vi "HFRR ADV v041.vi"() -> ()   [LabVIEW 2025] (continued)
          }
        }
        n1338 = local write "CAMERA ROI MAX TEMP"(TRUE ("CAMERA ROI MAX TEMP")) -> ()
      }
      frame "Adv Scar" {
        n1339 = local read "CAMERA ROI MIN TEMP"() -> (w1648:bool)
        n1340 = case shown="True" "LIVE FEED MAX TEMP" {
          selector: "LIVE FEED MAX TEMP" -> [_ w1669]
          frame False {
          }
          frame True {
            n1341 = Not(x=w1669) -> (.not. x?=w1668:bool)
            n1342 = local write "LIVE FEED MAX TEMP"(w1668) -> ()
            n1343 = call "CAMERA LIVE FEED FGV.vi"("Enum - Menu"=CAMERA_LIVE_FEED_ENUM."CAMERA RESTORE") -> ("error out"=w1659:errorcluster)  [unwired: 9 in, 1 out]
            n1344 = Type Cast(type=30, x=0) -> (*(type *) &x=w1663:i32)
            n1345 = Add(x=w1663, y=48) -> (x+y=w1664:i32)
            n1346 = call "CAMERA LIVE FEED FGV.vi"("Enum - Menu"=CAMERA_LIVE_FEED_ENUM."CAMERA MODE SET", "error in (no error)"=w1659, "CAMERA MODE"=w1664) -> ("error out"=w1656:errorcluster)  [unwired: 7 in, 1 out]
            n1347 = call "CAMERA LIVE FEED FGV.vi"("Enum - Menu"=CAMERA_LIVE_FEED_ENUM."CAMERA GRAY", "error in (no error)"=w1656) -> ("error out"=w1655:errorcluster)  [unwired: 8 in, 1 out]
            n1348 = call "LIST FILE NAMES.vi"("error in (no error)"=w1655) -> ("error out"=w1665:errorcluster, "filenames"=w1666:string[])  [unwired: 9 in]
            n1349 = property on="FILE 3" class="CmbBox"(error in=w1665, "Strings[]"=w1666) -> ()  [unwired: 1 in, 2 out]
          }
        }
        n1350 = case shown="True" w1648 {
          selector: w1648 -> [_ w1654]
          frame False {
          }
          frame True {
            n1351 = Not(x=w1654) -> (.not. x?=w1653:bool)
            n1352 = local write "CAMERA ROI MIN TEMP"(w1653) -> ()
            n1353 = call "IMAGE ANALYSIS.vi"("Enum"=POST_ANALYSIS_ENUM."MINIMIZE UI") -> ()  [unwired: 9 in, 2 out]
          }
        }
        n1354 = local write "CAMERA ROI MAX TEMP"(TRUE ("CAMERA ROI MAX TEMP")) -> ()
        "LIVE FEED MIN TEMP" <- TRUE ("LIVE FEED MIN TEMP")
      }
      frame "Adv Scar Report" {
        n1355 = local read "CAMERA ROI MAX TEMP"() -> (w1670:bool)
        n1356 = local read "LIVE FEED MIN TEMP"() -> (w1672:bool)
        n1357 = local write "LIVE FEED MAX TEMP"(TRUE ("LIVE FEED MAX TEMP")) -> ()
        n1358 = case shown="True" w1672 {
          selector: w1672 -> [_ w1681]
          frame False {
          }
          frame True {
            n1359 = Not(x=w1681) -> (.not. x?=w1680:bool)
            n1360 = local write "LIVE FEED MIN TEMP"(w1680) -> ()
            n1361 = call "CAMERA LIVE FEED FGV.vi"("Enum - Menu"=CAMERA_LIVE_FEED_ENUM."CAMERA MINIMIZE") -> ()  [unwired: 9 in, 2 out]
          }
        }
        n1362 = case shown="True" w1670 {
          selector: w1670 -> [_ w1678]
          frame False {
          }
          frame True {
            n1363 = Not(x=w1678) -> (.not. x?=w1676:bool)
            n1364 = local write "CAMERA ROI MAX TEMP"(w1676) -> ()
            n1365 = call "IMAGE ANALYSIS.vi"("Enum"=POST_ANALYSIS_ENUM."SHOW UI") -> ("error out"=w1675:errorcluster)  [unwired: 9 in, 1 out]
            n1366 = call "LIST FILE NAMES.vi"("error in (no error)"=w1675) -> ("filenames"=w1674:string[])  [unwired: 9 in, 1 out]
            n1367 = property on="Test File List :" class="CmbBox"("Strings[]"=w1674) -> ()  [unwired: 2 in, 2 out]
          }
        }
        n1368 = local write "CAMERA ROI MIN TEMP"(TRUE ("CAMERA ROI MIN TEMP")) -> ()
      }
      frame "Compare Files" {
        n1369 = local read "LIVE FEED MIN TEMP"() -> (w1684:bool)
        n1370 = local write "LIVE FEED MAX TEMP"(TRUE ("LIVE FEED MAX TEMP")) -> ()
        n1371 = local read "CAMERA ROI MIN TEMP"() -> (w1682:bool)
        n1372 = case shown="True" w1684 {
          selector: w1684 -> [_ w1691]
          frame False {
          }
          frame True {
            n1373 = Not(x=w1691) -> (.not. x?=w1690:bool)
            n1374 = local write "LIVE FEED MIN TEMP"(w1690) -> ()
            n1375 = call "CAMERA LIVE FEED FGV.vi"("Enum - Menu"=CAMERA_LIVE_FEED_ENUM."CAMERA MINIMIZE") -> ()  [unwired: 9 in, 2 out]
          }
        }
        n1376 = case shown="True" w1682 {
          selector: w1682 -> [_ w1688]
          frame False {
          }
          frame True {
            n1377 = Not(x=w1688) -> (.not. x?=w1687:bool)
            n1378 = local write "CAMERA ROI MIN TEMP"(w1687) -> ()
            n1379 = call "IMAGE ANALYSIS.vi"("Enum"=POST_ANALYSIS_ENUM."MINIMIZE UI") -> ()  [unwired: 9 in, 2 out]
          }
        }
        n1380 = local write "CAMERA ROI MAX TEMP"(TRUE ("CAMERA ROI MAX TEMP")) -> ()
      }
      frame "About" {
        n1381 = local read "LIVE FEED MIN TEMP"() -> (w1694:bool)
        n1382 = local write "LIVE FEED MAX TEMP"(TRUE ("LIVE FEED MAX TEMP")) -> ()
        n1383 = local read "CAMERA ROI MIN TEMP"() -> (w1693:bool)
        n1384 = case shown="True" w1694 {
          selector: w1694 -> [_ w1701]
          frame False {
          }
          frame True {
            n1385 = Not(x=w1701) -> (.not. x?=w1700:bool)
            n1386 = local write "LIVE FEED MIN TEMP"(w1700) -> ()
            n1387 = call "CAMERA LIVE FEED FGV.vi"("Enum - Menu"=CAMERA_LIVE_FEED_ENUM."CAMERA MINIMIZE") -> ()  [unwired: 9 in, 2 out]
          }
        }
        n1388 = case shown="True" w1693 {
          selector: w1693 -> [_ w1698]
          frame False {
          }
          frame True {
            n1389 = Not(x=w1698) -> (.not. x?=w1697:bool)
            n1390 = local write "CAMERA ROI MIN TEMP"(w1697) -> ()
            n1391 = call "IMAGE ANALYSIS.vi"("Enum"=POST_ANALYSIS_ENUM."MINIMIZE UI") -> ()  [unwired: 9 in, 2 out]
          }
        }
        n1392 = local write "CAMERA ROI MAX TEMP"(TRUE ("CAMERA ROI MIN TEMP")) -> ()
      }
      frame "Advance" {
        n1393 = local read "LIVE FEED MIN TEMP"() -> (w1704:bool)
        n1394 = local write "LIVE FEED MAX TEMP"(TRUE ("LIVE FEED MAX TEMP")) -> ()
        n1395 = local read "CAMERA ROI MIN TEMP"() -> (w1702:bool)
        n1396 = case shown="True" w1704 {
          selector: w1704 -> [_ w1711]
          frame False {
          }
          frame True {
            n1397 = Not(x=w1711) -> (.not. x?=w1710:bool)
            n1398 = local write "LIVE FEED MIN TEMP"(w1710) -> ()
            n1399 = call "CAMERA LIVE FEED FGV.vi"("Enum - Menu"=CAMERA_LIVE_FEED_ENUM."CAMERA MINIMIZE") -> ()  [unwired: 9 in, 2 out]
          }
        }
        n1400 = local write "CAMERA ROI MAX TEMP"(TRUE ("CAMERA ROI MAX TEMP")) -> ()
        n1401 = case shown="True" w1702 {
          selector: w1702 -> [_ w1708]
          frame False {
          }
          frame True {
            n1402 = Not(x=w1708) -> (.not. x?=w1707:bool)
            n1403 = local write "CAMERA ROI MIN TEMP"(w1707) -> ()
            n1404 = call "IMAGE ANALYSIS.vi"("Enum"=POST_ANALYSIS_ENUM."MINIMIZE UI") -> ()  [unwired: 9 in, 2 out]
          }
        }
      }
      frame "Mooha" {
        n1405 = local read "LIVE FEED MIN TEMP"() -> (w1714:bool)
        n1406 = local write "LIVE FEED MAX TEMP"(TRUE ("LIVE FEED MAX TEMP")) -> ()
        n1407 = local read "CAMERA ROI MIN TEMP"() -> (w1712:bool)
        n1408 = case shown="True" w1714 {
          selector: w1714 -> [_ w1721]
          frame False {
          }
          frame True {
            n1409 = Not(x=w1721) -> (.not. x?=w1720:bool)
            n1410 = local write "LIVE FEED MIN TEMP"(w1720) -> ()
            n1411 = call "CAMERA LIVE FEED FGV.vi"("Enum - Menu"=CAMERA_LIVE_FEED_ENUM."CAMERA MINIMIZE") -> ()  [unwired: 9 in, 2 out]
          }
        }
        n1412 = local write "CAMERA ROI MAX TEMP"(TRUE ("CAMERA ROI MAX TEMP")) -> ()
        n1413 = case shown="True" w1712 {
          selector: w1712 -> [_ w1718]
          frame False {
          }
          frame True {
            n1414 = Not(x=w1718) -> (.not. x?=w1717:bool)
            n1415 = local write "CAMERA ROI MIN TEMP"(w1717) -> ()
            n1416 = call "IMAGE ANALYSIS.vi"("Enum"=POST_ANALYSIS_ENUM."MINIMIZE UI") -> ()  [unwired: 9 in, 2 out]
          }
        }
      }
    }
    n1417 = local read "Auto Start Test"() -> (w1459:bool)
    n1418 = case shown="True" "sign in temp" {
      frame False {
      }
      frame True {
        w1494 = 1 ("y")
        n1419 = local read "USERNAME"() -> (w1500:string)
        n1420 = local read "USER ID"() -> (w1497:string)
        n1421 = call <vilib>:"Trim Whitespace.vi"("string"=w1500) -> ("trimmed string"=w1499:string)  [unwired: 1 in]
        n1422 = call <vilib>:"Trim Whitespace.vi"("string"=w1497) -> ("trimmed string"=w1498:string)  [unwired: 1 in]
        n1423 = String Length(string=w1499) -> (length=w1496:i32)
        n1424 = String Length(string=w1498) -> (length=w1495:i32)
        n1425 = Greater?(x=w1496, y=w1494) -> (0:w1493:bool)
        n1426 = Greater?(x=w1495, y=w1494) -> (0:w1492:bool)
        n1427 = And(x=w1493, y=w1492) -> (x .and. y?=w1491:bool)
        n1428 = case shown="True" w1491 {
          frame False {
            n1429 = property on="Sign In" class="Bool (strict)"("DisabledEnum"=T19."Disabled" ("Disabled")) -> ()  [unwired: 2 in, 2 out]
          }
          frame True {
            n1430 = property on="Sign In" class="Bool (strict)"("DisabledEnum"=T19."Enabled" ("Disabled")) -> ()  [unwired: 2 in, 2 out]
          }
        }
      }
    }
    n1431 = local read "Air Temperature"() -> (w1476:bool)
    n1432 = local read "Coefficient Of Friction"() -> (w1477:bool)
    n1433 = case shown="False" w1459 {
      frame False {
        n1434 = local read "Auto stop temp"() -> (w1488:bool)
        n1435 = case shown="True" w1488 {
          frame False {
          }
          frame True {
            n1436 = local write "Auto Start Temp"(FALSE ("Auto Start Temp")) -> ()
          }
        }
      }
      frame True {
        "Auto stop temp" <- TRUE ("Auto stop temp")
      }
    }
    n1437 = local read "Humidity"() -> (w1475:bool)
    n1438 = case shown="\"HOME\"" w1485 {
      frame "HOME" {
        n1439 = local write "main tab sub"(enum32{"Page 1", "Page 2"}."Page 1" ("main tab sub")) -> ()
      }
      frame Default {
        n1440 = local write "main tab sub"(enum32{"Page 1", "Page 2"}."Page 2" ("main tab sub")) -> ()
      }
    }
    n1441 = case shown="True" w1484 {
      selector: w1484 -> [_ w1836]
      frame False {
      }
      frame True {
        n1442 = Not(x=w1836) -> (.not. x?=w1835:bool)
        n1443 = local write "Sign In"(w1835) -> ()
        n1444 = local write "Main Dashboard Buttons"(T26."Test Setup" ("Main Dashboard Buttons")) -> ()
      }
    }
    n1445 = case shown="\"Numeric Display\", Default" "Num/Graph" {
      frame "Numeric Display", Default {
        n1446 = property on="Single/Multiple" class="RadioBtnsControl (strict)"("Visible"=FALSE) -> ()  [unwired: 2 in, 2 out]
        n1447 = property on="Single - Graph" class="Ring (strict)"("Visible"=FALSE) -> ()  [unwired: 2 in, 2 out]
        n1448 = local write "Main Tab Display"(T4."Dashboard 1" ("Main Tab Display")) -> ()
      }
      frame "Graph Display" {
        n1449 = property on="Single/Multiple" class="RadioBtnsControl (strict)"("Visible"=TRUE) -> ()  [unwired: 2 in, 2 out]
        n1450 = case shown="\"Multiple\"" "Single/Multiple" {
          frame "Single ", Default {
            n1451 = property on="Single - Graph" class="Ring (strict)"("Visible"=TRUE) -> ()  [unwired: 2 in, 2 out]
            n1452 = local write "Main Tab Display"(T4."Dashboard 3" ("Main Tab Display")) -> ()
          }
          frame "Multiple" {
            n1453 = property on="Single - Graph" class="Ring (strict)"("Visible"=FALSE) -> ()  [unwired: 2 in, 2 out]
            n1454 = local write "Main Tab Display"(T4."Dashboard 2" ("Main Tab Display")) -> ()
          }
        }
      }
    }
    n1455 = local read "Stroke"() -> (w1474:bool)
    n1456 = local read "USERNAME"() -> (w1479:string)
    n1457 = case shown="True" w1477 {
      selector: w1477 -> [_ w1761]
      frame False {
      }
      frame True {
        n1458 = Not(x=w1761) -> (.not. x?=w1760:bool)
        n1459 = local write "Coefficient Of Friction"(w1760) -> ()
        n1460 = local write "Tab Control 2"(T6."Coefficient Of Friction" ("Tab Control 2")) -> ()
      }
    }
    n1461 = case shown="True" w1476 {
      selector: w1476 -> [_ w1758]
      frame False {
      }
      frame True {
        n1462 = Not(x=w1758) -> (.not. x?=w1756:bool)
        n1463 = local write "Air Temperature"(w1756) -> ()
        n1464 = local write "Tab Control 2"(T6."Air Temperature" ("Tab Control 2")) -> ()
      }
    }
    n1465 = case shown="True" w1474 {
      selector: w1474 -> [_ w1752]
      frame False {
      }
      frame True {
        n1466 = Not(x=w1752) -> (.not. x?=w1750:bool)
        n1467 = local write "Stroke"(w1750) -> ()
        n1468 = local write "Tab Control 2"(T6."Stroke" ("Tab Control 2")) -> ()
      }
    }
    n1469 = local write "tested by"(w1479) -> ()
    n1470 = case shown="True" w1475 {
      selector: w1475 -> [_ w1755]
      frame False {
      }
      frame True {
        n1471 = Not(x=w1755) -> (.not. x?=w1753:bool)
        n1472 = local write "Humidity"(w1753) -> ()
        n1473 = local write "Tab Control 2"(T6."Humidity" ("Tab Control 2")) -> ()
      }
    }
    n1474 = case shown="\"Calibration\"" "Main Dashboard Buttons" {
      tunnel: [T2."HOME" ("Main Tab") T2."Test Setup" ("Main Tab") T2."Acquire" ("Main Tab") T2."Adv Scar" ("Main Tab") T2."Adv Scar Report" ("Main Tab") T2."Compare Files" ("Main Tab") T2."Calibration" ("Main Tab") T2."About" ("Main Tab") T2."Advance" ("Main Tab")] -> w1458
      frame "Home", Default {
      }
      frame "Test Setup" {
      }
      frame "Dashboard" {
      }
      frame "Imaging" {
      }
      frame "Report" {
      }
      frame "Analysis" {
      }
      frame "Calibration" {
      }
      frame "About" {
      }
      frame "Advance" {
      }
    }
    n1475 = Wait (ms)(milliseconds to wait=u32 100) -> ()  [unwired: 1 out]
    n1476 = local read "Main Tab Display"() -> (w1478:T4)
    n1477 = local write "Main Tab"(w1458) -> ()
    n1478 = case shown="\"Dashboard 3\"" w1478 {
      frame "Dashboard 1", Default {
        n1479 = property on="Reset Graph" class="Bool (strict)"("Visible"=FALSE) -> ()  [unwired: 2 in, 2 out]
      }
      frame "Dashboard 2" {
        n1480 = property on="Reset Graph" class="Bool (strict)"("Visible"=TRUE) -> ()  [unwired: 2 in, 2 out]
      }
      frame "Dashboard 3" {
        n1481 = property on="Reset Graph" class="Bool (strict)"("Visible"=TRUE) -> ()  [unwired: 2 in, 2 out]
      }
    }
    n1482 = local read "SCAR MEASURMENT"() -> (w1466:enum32{"Auto Scar", "Manual Scar"})
    n1483 = local read "Humidity"() -> (w1480:bool)
    n1484 = local read "Cap Live Image"() -> (w1463:bool)
    n1485 = local read "Sample Temperature"() -> (w1473:bool)
    n1486 = local read "Air Temp vs Humidity"() -> (w1471:bool)
    n1487 = local read "Frequency"() -> (w1472:bool)
    n1488 = case shown="False" w1480 {
      frame False {
        n1489 = local write "Humidity On Command"(TRUE ("Humidity On Command")) -> ()
        n1490 = case shown="True" "Humidity Off Command" {
          selector: "Humidity Off Command" -> [_ w1768]
          frame False {
          }
          frame True {
            n1491 = stacked-sequence {
              frame #0 {
                n1492 = local read "WriteHumidity"() -> (w1770:string[])
                n1493 = Insert Into Array(array=w1770, new element="R;1" ("new element/subarray")) -> (w1769:string[])  [unwired: 1 in]
                n1494 = local write "WriteHumidity"(w1769) -> ()
              }
              frame #1 {
                n1495 = Wait (ms)(milliseconds to wait=u32 500) -> ()  [unwired: 1 out]
              }
              frame #2 {
                n1496 = local read "WriteHumidity"() -> (w1774:string[])
                n1497 = local read "EVENT LOG"() -> (w1778:string)
                n1498 = call "Event Log.vi"("Content"="Humidity Control Off" ("string"), "EVENT LOG"=w1778) -> ("EVENT LOG"=w1779:string)  [unwired: 8 in, 1 out]
                n1499 = local write "EVENT LOG"(w1779) -> ()
                n1500 = Insert Into Array(array=w1774, new element="R;1" ("new element/subarray")) -> (w1775:string[])  [unwired: 1 in]
                n1501 = local write "WriteHumidity"(w1775) -> ()
                n1502 = local write "Humidity 2"(TRUE ("Humidity")) -> ()
              }
            }
            n1503 = Not(x=w1768) -> (.not. x?=w1767:bool)
            n1504 = local write "Humidity Off Command"(w1767) -> ()
          }
        }
      }
      frame True {
        n1505 = local write "Humidity Off Command"(TRUE ("Humidity Off Command")) -> ()
        n1506 = case shown="False" "Humidity On Command" {
          selector: "Humidity On Command" -> [_ w1783]
          frame False {
          }
          frame True {
            n1507 = stacked-sequence {
              frame #0 {
                n1508 = local read "Set Rh"() -> (w1789:dbl)
                n1509 = local read "WriteHumidity"() -> (w1785:string[])
                n1510 = Number To Fractional String(number=w1789, precision (6)=i16 2) -> (F-format string=w1790:string)  [unwired: 2 in]
                n1511 = Concatenate Strings("M;" ("new element/subarray"), w1790) -> (w1788:string)
                n1512 = Insert Into Array(array=w1785, new element=w1788) -> (w1784:string[])  [unwired: 1 in]
                n1513 = local write "WriteHumidity"(w1784) -> ()
              }
              frame #1 {
                n1514 = Wait (ms)(milliseconds to wait=u32 500) -> ()  [unwired: 1 out]
              }
              frame #2 {
                n1515 = local read "WriteHumidity"() -> (w1793:string[])
                n1516 = local read "Set Rh"() -> (w1797:dbl)
                n1517 = Number To Fractional String(number=w1797, precision (6)=i16 2) -> (F-format string=w1798:string)  [unwired: 2 in]
                n1518 = Concatenate Strings("M;" ("new element/subarray"), w1798) -> (w1796:string)
                n1519 = Insert Into Array(array=w1793, new element=w1796) -> (w1792:string[])  [unwired: 1 in]
                n1520 = local write "WriteHumidity"(w1792) -> ()
              }
              frame #3 {
                n1521 = Wait (ms)(milliseconds to wait=u32 500) -> ()  [unwired: 1 out]
              }
              frame #4 {
                (unwired) "% RH" ("string")
                (unwired) i16 2 ("precision (6)")
                (unwired) "M;" ("new element/subarray")
                n1522 = local read "Set Rh"() -> (w1807:dbl)
                n1523 = local read "WriteHumidity"() -> (w1800:string[])
                n1524 = Number To Fractional String(number=w1807, precision (6)=i16 2) -> (F-format string=w1804:string)  [unwired: 2 in]
                n1525 = Concatenate Strings("M;" ("new element/subarray"), w1804) -> (w1808:string)
                n1526 = Concatenate Strings("Humidity Set to : " ("string"), w1804, "% RH" ("string")) -> (w1802:string)
                n1527 = Insert Into Array(array=w1800, new element=w1808) -> (w1801:string[])  [unwired: 1 in]
                n1528 = disable-structure shown="Enabled" {
                  frame Enabled {
                    n1529 = local read "EVENT LOG"() -> (w1811:string)
                    n1530 = call "Event Log.vi"("Content"="Humidity Control On", "EVENT LOG"=w1811) -> ("EVENT LOG"=w1812:string)  [unwired: 8 in, 1 out]
                    n1531 = local write "EVENT LOG"(w1812) -> ()
                  }
                  frame Disabled {
                  }
                }
                n1532 = disable-structure shown="Enabled" {
                  disable-tunnel: w1802 -> [_ _]
                  frame Enabled {
                    n1533 = local read "EVENT LOG"() -> (w1814:string)
                    n1534 = call "Event Log.vi"("Content"="Humidity Control On", "EVENT LOG"=w1814) -> ("EVENT LOG"=w1815:string)  [unwired: 8 in, 1 out]
                    n1535 = local write "EVENT LOG"(w1815) -> ()
                  }
                  frame Disabled {
                  }
                }
                n1536 = local write "WriteHumidity"(w1801) -> ()
              }
            }
            n1537 = Not(x=w1783) -> (.not. x?=w1782:bool)
            n1538 = local write "Humidity On Command"(w1782) -> ()
          }
        }
      }
    }
    n1539 = Equal?(x=w1466, y=enum32{"Auto Scar", "Manual Scar"}."Auto Scar" ("SCAR MEASURMENT")) -> (x = y?=w1462:bool)
    n1540 = local read "TEST STANDARD"() -> (w1469:T3)
    n1541 = And(x=w1463, y=w1462) -> (x .and. y?=w1464:bool)
    n1542 = case shown="True" w1464 {
      selector: w1464 -> [_ w1567]
      tunnel: errorcluster {"status"=FALSE, "code"=0, "source"=""} ("error in (no error) 3") -> [_ w1568]
      frame False {
      }
      frame True {
        n1543 = stacked-sequence {
          tunnel: w1568 -> [_ _ _ _ _ _ _ w1616]
          tunnel: w1567 -> [_ _ _ _ _ w1597 _ _]
          frame #0 {
            n1544 = call "CAMERA LIVE FEED FGV.vi"("Enum - Menu"=CAMERA_LIVE_FEED_ENUM."CAMERA MINIMIZE") -> ()  [unwired: 9 in, 2 out]
          }
          frame #1 {
            n1545 = property on="Auto Scar Check  2" class="Clust (strict)"("Visible"=TRUE) -> ()  [unwired: 2 in, 2 out]
          }
          frame #2 {
            n1546 = String To Path(string="C:\\LAB-IQ\\Image Calibrate v01.dcf") -> (path=w1573:path)
            n1547 = Open/Create/Replace File ("Open File")(file path (use dialog)=w1573) -> (refnum out=w1574:refnum<file>)  [unwired: 5 in, 2 out]
            n1548 = for {
              N: 4 -> [_]
              tunnel: w1574 -> [w1580]
              i -> [w1576]
              n1549 = Read from Text File ("Read File")(file (use dialog)=w1580) -> (text=w1581:string)  [unwired: 3 in, 3 out]
              n1550 = String Subset(string=w1581, offset (0)=6, length (rest)=10 ("length (rest)")) -> (substring=w1577:string)
              n1551 = Fract/Exp String To Number(string=w1577) -> (number=w1575:dbl)  [unwired: 3 in, 1 out]
              n1552 = case shown="0" w1576 {
                tunnel: w1575 -> [w1582 w1583 _ w1584 _]
                frame 0 {
                  "5x Gain" <- w1582
                }
                frame 1 {
                  "10x Gain" <- w1583
                }
                frame 2 {
                }
                frame 3 {
                  "100x gain" <- w1584
                }
                frame 4, Default {
                }
              }
            }
          }
          frame #3 {
            n1553 = local read "FILE 3"() -> (w1590:string)
            n1554 = call <vilib>:"Trim Whitespace.vi"("string"="C:\\LAB-IQ\\images\\") -> ("trimmed string"=w1592:string)  [unwired: 1 in]
            n1555 = String To Path(string=w1592) -> (path=w1591:path)
            n1556 = Concatenate Strings(w1590, ".png" ("string")) -> (w1589:string)
            n1557 = Build Path(base path=w1591, name or relative path=w1589) -> (appended path=w1587:path)
            "Image path" <- w1587
            n1558 = Path To String(path=w1587) -> (string=w1586:string)
            n1559 = call "CAMERA LIVE FEED FGV.vi"("Enum - Menu"=CAMERA_LIVE_FEED_ENUM."CAMERA SAVE", "Image Path"=w1586) -> ()  [unwired: 8 in, 2 out]
          }
          frame #4 {
            n1560 = One Button Dialog(message="Image saved successfully") -> ()  [unwired: 1 in, 1 out]
          }
          frame #5 {
            n1561 = local read "TEST STANDARD"() -> (w1596:T3)
            n1562 = local read "Magnification len live scar"() -> (w1608:string)
            n1563 = Not(x=w1597) -> (.not. x?=w1598:bool)
            n1564 = local write "Cap Live Image"(w1598) -> ()
            n1565 = case shown="\"ISO 12156\"" w1596 {
              tunnel: ["ASTM D6079" "ISO 12156"] -> w1595
              frame "ASTM D6079", Default {
              }
              frame "ISO 12156" {
              }
            }
            n1566 = case shown="\"5x\", Default" w1608 {
              tunnel: [w1611 w1612] -> w1607
              frame "5x", Default {
                n1567 = local read "5x Gain"() -> (w1611:dbl)
              }
              frame "10x" {
                # "5x"
                n1568 = local read "10x Gain"() -> (w1612:dbl)
              }
            }
            n1569 = local read "Image path"() -> (w1606:path)
            n1570 = local read "FILE 3"() -> (w1599:string)
            n1571 = call "EDGE DETCTION.vi"("GAIN VALUE"=w1607, "Image Path"=w1606) -> ("error out"=w1605:errorcluster, "return value"=w1604:cluster{string, string, dbl, dbl, dbl})  [unwired: 8 in]
            n1572 = Bundle By Name(cluster=T27 {"File Name"="", "Test Method"="", "Operator"="", "Fuel Description"="", "Date and time"=""} ("Main Ref"), "File Name"=w1599, "Test Method"=w1595) -> (w1600:T27)
            n1573 = call "duf file read.vi"("error in (no error)"=w1605, "Main Ref"=w1600) -> ("error out"=w1603:errorcluster, "Main Ref 2"=w1601:T27)  [unwired: 8 in]
            n1574 = call "EDGE DETECTION REPORT.vi"("error in (no error)"=w1603, "return value 2"=w1604, "Main Ref"=w1601) -> ()  [unwired: 8 in, 1 out]
          }
          frame #6 {
            n1575 = property on="Auto Scar Check  2" class="Clust (strict)"("Visible"=FALSE) -> ()  [unwired: 2 in, 2 out]
          }
          frame #7 {
            n1576 = call "CAMERA LIVE FEED FGV.vi"("Enum - Menu"=CAMERA_LIVE_FEED_ENUM."CAMERA MINIMIZE", "error in (no error)"=w1616) -> ()  [unwired: 8 in, 2 out]
            n1577 = local write "Main Dashboard Buttons"(T1."Home" ("Main Dashboard Buttons")) -> ()
            n1578 = local write "Main Tab"(T2."HOME" ("Main Tab")) -> ()
          }
        }
      }
    }
    n1579 = local read "Heater Button"() -> (w1470:bool)
    n1580 = case shown="True" w1472 {
      selector: w1472 -> [_ w1746]
      frame False {
      }
      frame True {
        n1581 = Not(x=w1746) -> (.not. x?=w1744:bool)
        n1582 = local write "Frequency"(w1744) -> ()
        n1583 = local write "Tab Control 2"(T6."Frequency" ("Tab Control 2")) -> ()
      }
    }
    n1584 = case shown="True" w1471 {
      selector: w1471 -> [_ w1743]
      frame False {
      }
      frame True {
        n1585 = Not(x=w1743) -> (.not. x?=w1741:bool)
        n1586 = local write "Air Temp vs Humidity"(w1741) -> ()
        n1587 = local write "Tab Control 2"(T6."Air Temp vs Rh" ("Tab Control 2")) -> ()
      }
    }
    n1588 = case shown="True" w1473 {
      selector: w1473 -> [_ w1749]
      frame False {
      }
      frame True {
        n1589 = Not(x=w1749) -> (.not. x?=w1747:bool)
        n1590 = local write "Sample Temperature"(w1747) -> ()
        n1591 = local write "Tab Control 2"(T6."Sample Temperature" ("Tab Control 2")) -> ()
      }
    }
    n1592 = case shown="\"Custom\"" w1469 {
      frame "ASTM D6079", Default {
        w1722 = "ASTM D6079 TEST CONDITIONS" ("Standard 2")
        n1593 = local write "Standard 2"(w1722) -> ()
        n1594 = local write "Standard"(w1722) -> ()
      }
      frame "ISO 12156" {
        w1723 = "ISO 12156 TEST CONDITIONS" ("Standard 2")
        n1595 = local write "Standard 2"(w1723) -> ()
        n1596 = local write "Standard"(w1723) -> ()
      }
      frame "CEC F-096-A-06" {
        w1724 = "CEC F-096-A-06 TEST CONDITIONS" ("Standard 2")
        n1597 = local write "Standard 2"(w1724) -> ()
        n1598 = local write "Standard"(w1724) -> ()
      }
      frame "Custom" {
        w1725 = "CUSTOM TEST CONDITIONS" ("Standard 2")
        n1599 = local write "Standard 2"(w1725) -> ()
        n1600 = local write "Standard"(w1725) -> ()
      }
    }
    n1601 = case shown="True" w1470 {
      frame False {
        n1602 = local write "Temperature On Command"(TRUE ("Temperature On Command")) -> ()
        n1603 = case shown="True" "Temperature Off Command" {
          selector: "Temperature Off Command" -> [_ w1729]
          frame False {
          }
          frame True {
            n1604 = Not(x=w1729) -> (.not. x?=w1728:bool)
            n1605 = local read "EVENT LOG"() -> (w1732:string)
            n1606 = local write "Temperature Off Command"(w1728) -> ()
            n1607 = call "Event Log.vi"("Content"="Heater Off", "EVENT LOG"=w1732) -> ("EVENT LOG"=w1731:string)  [unwired: 8 in, 1 out]
            n1608 = local write "EVENT LOG"(w1731) -> ()
          }
        }
      }
      frame True {
        n1609 = local write "Temperature Off Command"(TRUE ("Temperature Off Command")) -> ()
        n1610 = case shown="True" "Temperature On Command" {
          selector: "Temperature On Command" -> [_ w1736]
          frame False {
          }
          frame True {
            n1611 = Not(x=w1736) -> (.not. x?=w1735:bool)
            n1612 = local write "Temperature On Command"(w1735) -> ()
            n1613 = disable-structure shown="Enabled" {
              disable-tunnel: "Heater On" -> [w1738 _]
              frame Enabled {
                n1614 = local read "EVENT LOG"() -> (w1739:string)
                n1615 = call "Event Log.vi"("Content"=w1738, "EVENT LOG"=w1739) -> ("EVENT LOG"=w1740:string)  [unwired: 8 in, 1 out]
                n1616 = local write "EVENT LOG"(w1740) -> ()
              }
              frame Disabled {
              }
            }
          }
        }
      }
    }
    n1617 = local read "Main Tab"() -> (w1461:T2)
    n1618 = case shown="\"About\"" w1461 {
      frame "HOME", Default {
        w1503 = T19."Enabled" ("Disabled")
        n1619 = local read "Service Password enable"() -> (w1505:bool)
        n1620 = property on="Imaging" class="Bool (strict)"("DisabledEnum"=w1503) -> ()  [unwired: 2 in, 2 out]
        n1621 = property on="Dashboard" class="Bool (strict)"("DisabledEnum"=w1503) -> ()  [unwired: 2 in, 2 out]
        n1622 = property on="Test Setup" class="Bool (strict)"("DisabledEnum"=w1503) -> ()  [unwired: 2 in, 2 out]
        n1623 = property on="Analysis" class="Bool (strict)"("DisabledEnum"=w1503) -> ()  [unwired: 2 in, 2 out]
        n1624 = property on="Home" class="Bool (strict)"("DisabledEnum"=w1503) -> ()  [unwired: 2 in, 2 out]
        n1625 = property on="Report" class="Bool (strict)"("DisabledEnum"=w1503) -> ()  [unwired: 2 in, 2 out]
        n1626 = property on="Main Dashboard Buttons" class="RadioBtnsControl (strict)"("DisabledEnum"=w1503) -> ()  [unwired: 2 in, 2 out]
        n1627 = property on="Calibration" class="Bool (strict)"("DisabledEnum"=w1503) -> ()  [unwired: 2 in, 2 out]
        n1628 = case shown="True" w1505 {
          tunnel: [T19."Disabled" ("Disabled") T19."Enabled" ("Disabled")] -> w1504
          frame False {
          }
          frame True {
          }
        }
        n1629 = property on="About" class="Bool (strict)"("DisabledEnum"=w1504) -> ()  [unwired: 2 in, 2 out]
      }
      frame "Test Setup" {
        w1510 = T19."Enabled" ("Disabled")
        n1630 = local read "Service Password enable"() -> (w1509:bool)
        n1631 = property on="Dashboard" class="Bool (strict)"("DisabledEnum"=T19."Disabled" ("Disabled")) -> ()  [unwired: 2 in, 2 out]
        n1632 = property on="Imaging" class="Bool (strict)"("DisabledEnum"=w1510) -> ()  [unwired: 2 in, 2 out]
        n1633 = property on="Analysis" class="Bool (strict)"("DisabledEnum"=w1510) -> ()  [unwired: 2 in, 2 out]
        n1634 = property on="Home" class="Bool (strict)"("DisabledEnum"=w1510) -> ()  [unwired: 2 in, 2 out]
        n1635 = property on="Report" class="Bool (strict)"("DisabledEnum"=w1510) -> ()  [unwired: 2 in, 2 out]
        n1636 = property on="Test Setup" class="Bool (strict)"("DisabledEnum"=w1510) -> ()  [unwired: 2 in, 2 out]
        n1637 = case shown="True" w1509 {
          tunnel: [T19."Disabled" ("Disabled") T19."Enabled" ("Disabled")] -> w1508
          frame False {
          }
          frame True {
          }
        }
        n1638 = property on="About" class="Bool (strict)"("DisabledEnum"=w1508) -> ()  [unwired: 2 in, 2 out]
      }
      frame "Adv Scar" {
        w1517 = T19."Enabled" ("Disabled")
        n1639 = property on="Dashboard" class="Bool (strict)"("DisabledEnum"=T19."Disabled" ("Disabled")) -> ()  [unwired: 2 in, 2 out]
        n1640 = property on="Imaging" class="Bool (strict)"("DisabledEnum"=w1517) -> ()  [unwired: 2 in, 2 out]
        n1641 = property on="Analysis" class="Bool (strict)"("DisabledEnum"=w1517) -> ()  [unwired: 2 in, 2 out]
        n1642 = property on="Home" class="Bool (strict)"("DisabledEnum"=w1517) -> ()  [unwired: 2 in, 2 out]
        n1643 = property on="Report" class="Bool (strict)"("DisabledEnum"=w1517) -> ()  [unwired: 2 in, 2 out]
        n1644 = property on="Test Setup" class="Bool (strict)"("DisabledEnum"=w1517) -> ()  [unwired: 2 in, 2 out]
        n1645 = local read "Service Password enable"() -> (w1515:bool)
        n1646 = case shown="True" w1515 {
          tunnel: [T19."Disabled" ("Disabled") T19."Enabled" ("Disabled")] -> w1514
          frame False {
          }
          frame True {
          }
        }
        n1647 = property on="About" class="Bool (strict)"("DisabledEnum"=w1514) -> ()  [unwired: 2 in, 2 out]
      }
      frame "Calibration" {
        w1520 = T19."Enabled" ("Disabled")
        n1648 = property on="Dashboard" class="Bool (strict)"("DisabledEnum"=T19."Disabled" ("Disabled")) -> ()  [unwired: 2 in, 2 out]
        n1649 = property on="Imaging" class="Bool (strict)"("DisabledEnum"=w1520) -> ()  [unwired: 2 in, 2 out]
        n1650 = property on="Analysis" class="Bool (strict)"("DisabledEnum"=w1520) -> ()  [unwired: 2 in, 2 out]
        n1651 = property on="Home" class="Bool (strict)"("DisabledEnum"=w1520) -> ()  [unwired: 2 in, 2 out]
        n1652 = property on="Report" class="Bool (strict)"("DisabledEnum"=w1520) -> ()  [unwired: 2 in, 2 out]
        n1653 = property on="Test Setup" class="Bool (strict)"("DisabledEnum"=w1520) -> ()  [unwired: 2 in, 2 out]
        n1654 = local read "Service Password enable"() -> (w1522:bool)
        n1655 = property on="Calibration" class="Bool (strict)"("DisabledEnum"=w1520) -> ()  [unwired: 2 in, 2 out]
        n1656 = case shown="True" w1522 {
          tunnel: [T19."Disabled" ("Disabled") T19."Enabled" ("Disabled")] -> w1521
          frame False {
          }
          frame True {
          }
        }
        n1657 = property on="About" class="Bool (strict)"("DisabledEnum"=w1521) -> ()  [unwired: 2 in, 2 out]
      }
      frame "Adv Scar Report" {
        w1528 = T19."Enabled" ("Disabled")
        n1658 = property on="Dashboard" class="Bool (strict)"("DisabledEnum"=T19."Disabled" ("Disabled")) -> ()  [unwired: 2 in, 2 out]
        n1659 = property on="Imaging" class="Bool (strict)"("DisabledEnum"=w1528) -> ()  [unwired: 2 in, 2 out]
        n1660 = property on="Analysis" class="Bool (strict)"("DisabledEnum"=w1528) -> ()  [unwired: 2 in, 2 out]
        n1661 = property on="Home" class="Bool (strict)"("DisabledEnum"=w1528) -> ()  [unwired: 2 in, 2 out]
        n1662 = property on="Report" class="Bool (strict)"("DisabledEnum"=w1528) -> ()  [unwired: 2 in, 2 out]
        n1663 = property on="Test Setup" class="Bool (strict)"("DisabledEnum"=w1528) -> ()  [unwired: 2 in, 2 out]
        n1664 = local read "Service Password enable"() -> (w1527:bool)
        n1665 = case shown="True" w1527 {
          tunnel: [T19."Disabled" ("Disabled") T19."Enabled" ("Disabled")] -> w1526
          frame False {
          }
          frame True {
          }
        }
        n1666 = property on="About" class="Bool (strict)"("DisabledEnum"=w1526) -> ()  [unwired: 2 in, 2 out]
      }
      frame "Compare Files" {
        w1534 = T19."Enabled" ("Disabled")
        n1667 = local read "Service Password enable"() -> (w1533:bool)
        n1668 = property on="Dashboard" class="Bool (strict)"("DisabledEnum"=T19."Disabled" ("Disabled")) -> ()  [unwired: 2 in, 2 out]
        n1669 = property on="Imaging" class="Bool (strict)"("DisabledEnum"=w1534) -> ()  [unwired: 2 in, 2 out]
        n1670 = property on="Analysis" class="Bool (strict)"("DisabledEnum"=w1534) -> ()  [unwired: 2 in, 2 out]
        n1671 = property on="Home" class="Bool (strict)"("DisabledEnum"=w1534) -> ()  [unwired: 2 in, 2 out]
        n1672 = property on="Report" class="Bool (strict)"("DisabledEnum"=w1534) -> ()  [unwired: 2 in, 2 out]
        n1673 = property on="Test Setup" class="Bool (strict)"("DisabledEnum"=w1534) -> ()  [unwired: 2 in, 2 out]
        n1674 = case shown="True" w1533 {
          tunnel: [T19."Disabled" ("Disabled") T19."Enabled" ("Disabled")] -> w1532
          frame False {
          }
          frame True {
          }
        }
        n1675 = property on="About" class="Bool (strict)"("DisabledEnum"=w1532) -> ()  [unwired: 2 in, 2 out]
      }
      frame "Acquire" {
        n1676 = local read "Service Password enable"() -> (w1539:bool)
        n1677 = property on="Test Setup" class="Bool (strict)"("DisabledEnum"=T19."Disabled" ("Disabled")) -> ()  [unwired: 2 in, 2 out]
        n1678 = local read "Auto Start Test"() -> (w1541:bool)
        n1679 = local read "RUN"() -> (w1543:bool)
        n1680 = case shown="True" w1539 {
          tunnel: [T19."Disabled" ("Disabled") T19."Enabled" ("Disabled")] -> w1540
          frame False {
          }
          frame True {
          }
        }
        n1681 = Or(x=w1543, y=w1541) -> (x .or. y?=w1542:bool)
        n1682 = case shown="True" w1542 {
          tunnel: [T19."Enabled" ("Disabled") T19."Disabled" ("Disabled")] -> w1538
          frame False {
          }
          frame True {
          }
        }
        n1683 = property on="About" class="Bool (strict)"("DisabledEnum"=w1540) -> ()  [unwired: 2 in, 2 out]
        n1684 = property on="Imaging" class="Bool (strict)"("DisabledEnum"=w1538) -> ()  [unwired: 2 in, 2 out]
        n1685 = property on="Dashboard" class="Bool (strict)"("DisabledEnum"=w1538) -> ()  [unwired: 2 in, 2 out]
        n1686 = property on="Analysis" class="Bool (strict)"("DisabledEnum"=w1538) -> ()  [unwired: 2 in, 2 out]
        n1687 = property on="Home" class="Bool (strict)"("DisabledEnum"=w1538) -> ()  [unwired: 2 in, 2 out]
        n1688 = property on="Report" class="Bool (strict)"("DisabledEnum"=w1538) -> ()  [unwired: 2 in, 2 out]
        n1689 = property on="Calibration" class="Bool (strict)"("DisabledEnum"=w1538) -> ()  [unwired: 2 in, 2 out]
      }
      frame "About" {
        n1690 = local read "FILE"() -> (w1557:string)
        n1691 = local read "TEST FILE NAM,E SAVED"() -> (w1550:bool)
        n1692 = call <vilib>:"Trim Whitespace.vi"("string"=w1557) -> ("trimmed string"=w1556:string)  [unwired: 1 in]
        n1693 = local read "Auto Start Test"() -> (w1560:bool)
        n1694 = String Length(string=w1556) -> (length=w1555:i32)
        n1695 = Greater?(x=w1555, y=1) -> (0:w1552:bool)
        n1696 = And(x=w1552, y=w1550) -> (x .and. y?=w1551:bool)
        n1697 = local read "RUN"() -> (w1562:bool)
        n1698 = case shown="True" w1551 {
          tunnel: [T19."Disabled" ("Disabled") T19."Enabled" ("Disabled")] -> w1553
          frame False {
          }
          frame True {
          }
        }
        n1699 = Or(x=w1562, y=w1560) -> (x .or. y?=w1561:bool)
        n1700 = property on="About" class="Bool (strict)"("DisabledEnum"=T19."Enabled" ("Disabled")) -> ()  [unwired: 2 in, 2 out]
        n1701 = case shown="False" w1561 {
          tunnel: [T19."Enabled" ("Disabled") T19."Disabled" ("Disabled")] -> w1559
          frame False {
          }
          frame True {
          }
        }
        n1702 = property on="Dashboard" class="Bool (strict)"("DisabledEnum"=w1553) -> ()  [unwired: 2 in, 2 out]
        n1703 = property on="Test Setup" class="Bool (strict)"("DisabledEnum"=T19."Disabled" ("Disabled")) -> ()  [unwired: 2 in, 2 out]
        n1704 = property on="Imaging" class="Bool (strict)"("DisabledEnum"=w1559) -> ()  [unwired: 2 in, 2 out]
        n1705 = property on="Analysis" class="Bool (strict)"("DisabledEnum"=w1559) -> ()  [unwired: 2 in, 2 out]
        n1706 = property on="Home" class="Bool (strict)"("DisabledEnum"=w1559) -> ()  [unwired: 2 in, 2 out]
        n1707 = property on="Report" class="Bool (strict)"("DisabledEnum"=w1559) -> ()  [unwired: 2 in, 2 out]
      }
    }
    n1708 = local read "Quit"() -> (w1487:bool)
    "Single" <- "Single - Graph"
  }
  n1709 = disable-structure shown="Disabled" {
    disable-tunnel: [w1840 _] -> w44
    disable-tunnel: _ -> [w1839 _]
    frame Disabled {
      n1710 = while {
        tunnel: w1839 -> [_]
        tunnel: [w1841] -> w1840
        tunnel: [w1842] -> _
        i -> [w1842]
        stop <- w1841 stop-if-true
        w1858 = u16 10 items=["1.0"=10, "1.5"=15, "2.0"=20] ("stop bits (10: 1 bit)")
        n1711 = Wait (ms)(milliseconds to wait=u32 10) -> ()  [unwired: 1 out]
        n1712 = call-poly "VISA Configure Serial Port"("VISA resource name"=refnum<visa-resource-name> "ASRL1::INSTR" ("COM PORT"), "timeout (10sec)"=u32 10, "baud rate (9600)"=u32 57600, "data bits (8)"=u16 8, "stop bits (10: 1 bit)"=w1858) -> ("VISA resource name out"=w1844:refnum<visa-resource-name>, "error out"=w1853:errorcluster)  [unwired: 9 in]
        n1713 = VISA Read(VISA resource name=w1844, byte count=u32 2 ("byte count (0)")) -> (read buffer=w1852:string)  [unwired: 1 in, 3 out]
        n1714 = String Subset(string=w1852, offset (0)=0, length (rest)=2 ("length (rest)")) -> (substring=w1851:string)
        n1715 = Match Pattern(string=w1851, regular expression="<>") -> (offset past match=w1848:i32)  [unwired: 1 in, 3 out]
        n1716 = Greater Or Equal?(x=w1848, y=0) -> (x >= y?=w1843:bool)
        n1717 = case shown="True" w1843 {
          tunnel: w1844 -> [_ w1862]
          tunnel: w1853 -> [_ w1861]
          frame False {
          }
          frame True {
            n1718 = VISA Read(VISA resource name=w1862, byte count=u32 32 ("byte count (0)"), error in (no error)=w1861) -> (read buffer=w1860:string)  [unwired: 3 out]
            n1719 = String Subset(string=w1860, offset (0)=0, length (rest)=8 ("length (rest)")) -> (substring=w1864:string)
            n1720 = String Subset(string=w1860, offset (0)=8, length (rest)=8 ("length (rest)")) -> (substring=w1865:string)
            n1721 = Decimal String To Number(string=w1865) -> (number=w1872:i32)  [unwired: 2 in, 1 out]
            n1722 = Decimal String To Number(string=w1864) -> (number=w1868:i32)  [unwired: 2 in, 1 out]
            n1723 = Divide(x=w1872, y=10000) -> ()  [unwired: 1 out]
            n1724 = Divide(x=w1868, y=1000000) -> ()  [unwired: 1 out]
          }
        }
        n1725 = local read "Quit"() -> (w1841:bool)
      }
    }
    frame Enabled {
    }
  }
  n1726 = Tick Count (ms)() -> (millisecond timer value=w6:u32)
  n1727 = while {
    shift-right: [w1918] -> _
    shift-left: w8 -> [w1922]
    shift-right: [w1917] -> _
    shift-left: w7 -> [w1921]
    shift-right: [w1916] -> _
    shift-left: w8 -> [w1920]
    shift-right: [w1915] -> _
    shift-left: w7 -> [w1919]
    shift-right: [w1913] -> _
    shift-left: w6 -> [w1914]
    shift-right: [w1910] -> _
    shift-left: w5 -> [w1911]
    shift-right: [w1909] -> _
    shift-left: w5 -> [w1912]
    shift-right: [w1902] -> _
    shift-left: w5 -> [w1908]
    shift-right: [w1901] -> _
    shift-left: w5 -> [w1907]
    shift-right: [w1900] -> _
    shift-left: w5 -> [w1906]
    shift-right: [w1899] -> _
    shift-left: w5 -> [w1905]
    shift-right: [w1898] -> _
    shift-left: w5 -> [w1904]
    shift-right: [w1897] -> _
    shift-left: w5 -> [w1903]
    shift-right: [w1896] -> _
    shift-left: w5 -> [w1890]
    shift-right: [w1895] -> _
    shift-left: w5 -> [w1889]
    shift-right: [w1894] -> _
    shift-left: w5 -> [w1888]
    shift-right: [w1893] -> _
    shift-left: w5 -> [w1887]
    shift-right: [w1892] -> _
    shift-left: w5 -> [w1886]
    shift-right: [w1891] -> _
    shift-left: w5 -> [w1885]
    shift-right: [w1876] -> _
    shift-left: w5 -> [w1879]
    shift-right: [w1875] -> _
    shift-left: w5 -> [w1878]
    shift-right: [w1874] -> _
    shift-left: w5 -> [w1877]
    stop <- w1924 stop-if-true
    n1728 = local read "Read UNO"() -> (w1883:string)
    n1729 = local read "Error  2"() -> (w1923:errorcluster)
    n1730 = String Length(string=w1883) -> (length=w1882:i32)
    n1731 = call <vilib>:"Trim Whitespace.vi"("string"=w1883) -> ("trimmed string"=w1884:string)  [unwired: 1 in]
    n1732 = Greater Or Equal?(x=w1882, y=23) -> (x >= y?=w1880:bool)
    n1733 = case shown="No Error" w1923 {
      tunnel: w1922 -> [w1970 w2066]
      tunnel: w1921 -> [w1969 w2065]
      tunnel: w1920 -> [w1968 w2064]
      tunnel: w1919 -> [w1967 w2063]
      tunnel: [w1966 w2066] -> w1918
      tunnel: [w1965 w2065] -> w1917
      tunnel: [w1964 w2064] -> w1916
      tunnel: [w1963 w2063] -> w1915
      tunnel: w1914 -> [w1962 w2062]
      tunnel: [w1961 w2062] -> w1913
      tunnel: w1911 -> [w1960 w2061]
      tunnel: w1912 -> [w1959 w2060]
      tunnel: [w1958 w2061] -> w1910
      tunnel: [w1957 w2060] -> w1909
      tunnel: w1908 -> [w1956 w2059]
      tunnel: w1907 -> [w1955 w2058]
      tunnel: w1906 -> [w1954 w2057]
      tunnel: w1905 -> [w1953 w2056]
      tunnel: w1904 -> [w1952 w2055]
      tunnel: w1903 -> [w1951 w2054]
      tunnel: [w1950 w2059] -> w1902
      tunnel: [w1949 w2058] -> w1901
      tunnel: [w1948 w2057] -> w1900
      tunnel: [w1947 w2056] -> w1899
      tunnel: [w1946 w2055] -> w1898
      tunnel: [w1945 w2054] -> w1897
      tunnel: w1890 -> [w1944 w2053]
      tunnel: [w1943 w2053] -> w1896
      tunnel: [w1942 w2049] -> w1895
      tunnel: [w1941 w2048] -> w1894
      tunnel: [w1940 w2052] -> w1893
      tunnel: [w1939 w2051] -> w1892
      tunnel: [w1938 w2050] -> w1891
      tunnel: w1889 -> [w1937 w2052]
      tunnel: w1888 -> [w1936 w2051]
      tunnel: w1887 -> [w1935 w2050]
      tunnel: w1886 -> [w1934 w2049]
      tunnel: w1885 -> [w1933 w2048]
      tunnel: w1884 -> [w1932 _]
      tunnel: w1880 -> [w1931 _]
      tunnel: w1879 -> [w1930 w2047]
      tunnel: w1878 -> [w1929 w2046]
      tunnel: w1877 -> [w1928 w2045]
      tunnel: [w1927 w2047] -> w1876
      tunnel: [w1926 w2046] -> w1875
      tunnel: [w1925 w2045] -> w1874
      frame No Error {
        n1734 = case shown="True" w1931 {
          tunnel: w1970 -> [w1986 w2038]
          tunnel: w1969 -> [w1985 w2037]
          tunnel: w1968 -> [w1984 w2036]
          tunnel: w1967 -> [w1983 w2035]
          tunnel: [w1986 w2034] -> w1966
          tunnel: [w1985 w2033] -> w1965
          tunnel: [w1984 w2032] -> w1964
          tunnel: [w1983 w2031] -> w1963
          tunnel: w1962 -> [w1982 w2029]
          tunnel: [w1982 w2028] -> w1961
          tunnel: w1960 -> [w1981 w2027]
          tunnel: w1959 -> [w1980 w2026]
          tunnel: [w1981 w2025] -> w1958
          tunnel: [w1980 w2024] -> w1957
          tunnel: w1956 -> [w1979 w2023]
          tunnel: w1955 -> [w1978 w2022]
          tunnel: w1954 -> [w1977 w2021]
          tunnel: w1953 -> [w1976 w2020]
          tunnel: w1952 -> [w1975 w2019]
          tunnel: w1951 -> [w1974 w2018]
          tunnel: [w1979 w2017] -> w1950
          tunnel: [w1978 w2016] -> w1949
          tunnel: [w1977 w2015] -> w1948
          tunnel: [w1976 w2014] -> w1947
          tunnel: [w1975 w2013] -> w1946
          tunnel: [w1974 w2012] -> w1945
          tunnel: w1944 -> [w1992 w2011]
          tunnel: [w1992 w2010] -> w1943
          tunnel: [w1989 w2009] -> w1942
          tunnel: [w1988 w2008] -> w1941
          tunnel: [w1991 w2007] -> w1940
          tunnel: [w1987 w2006] -> w1939
          tunnel: [w1990 w2005] -> w1938
          tunnel: w1937 -> [w1991 w2004]
          tunnel: w1936 -> [w1990 w2003]
          tunnel: w1935 -> [w1989 w2002]
          tunnel: w1934 -> [w1988 w2001]
          tunnel: w1933 -> [w1987 w2000]
          tunnel: w1932 -> [_ w1999]
          tunnel: w1930 -> [w1973 w1998]
          tunnel: w1929 -> [w1972 w1997]
          tunnel: w1928 -> [w1971 w1996]
          tunnel: [w1973 w1995] -> w1927
          tunnel: [w1972 w1994] -> w1926
          tunnel: [w1971 w1993] -> w1925
          frame False {
          }
          frame True {
            n1735 = Tick Count (ms)() -> (millisecond timer value=w2030:u32)
            n1736 = String To Byte Array(string=w1999) -> (unsigned byte array=w2043:u8[])
            n1737 = Array Size(array=w2043) -> (size(s)=w2042:i32)
            n1738 = formula code="// --- INTERNAL VARIABLE DECLARATIONS ---\nint i = 0;\nint k = 0;\nint start_idx = -1;\nint end_idx = -1;\nint phase = 0;\nint sign0 = 1;\nint sign1 = 1;\nint ch0_val = 0;   \nint ch1_val = 0;   \nfloat ch0_raw = 0.0;\nfloat ch1_raw = 0.0;\nfloat temp0 = 0.0;\nfloat temp1 = 0.0;\nfloat ch0_clean = 0.0;\nfloat ch1_clean = 0.0;\n\nint valid_samples = 0; // FIX: Track if we actually parsed new data this window\nfloat max_allowed_bits = 8388607.0; // FIX: Change this to match your ADC max value\n\n// Temporal intermediate variables for calculation smoothing\nfloat raw_p2p_v = 0.0;\nfloat raw_friction = 0.0;\nfloat raw_cof = 0.0;\n\n// Temporal intermediate variables for Piezo voltage translations\nfloat piezo_min_v = 0.0;\nfloat piezo_max_v = 0.0;\n\n// Initialize output variables to current shift register states right away\nout_LVDT_Min_V = in_LVDT_Min_V;\nout_LVDT_Max_V = in_LVDT_Max_V;\nout_LVDT_P2P_V = in_LVDT_P2P_V;\nout_Piezo_P2P = in_Piezo_P2P;\nout_Friction_N = in_Friction_N;\nout_COF = in_COF;\nwindow_ready = 0;\n\n// --- STEP 1: PARSE EVERY STRING IN THE BYTE ARRAY ---\nif (array_size > 2) {\n    for (i = 0; i < array_size - 1; i++) {\n        if (raw_bytes[i] == 42) { // '*' character detected\n            start_idx = i;\n        }\n        \n        // Match standard delimiter sequence \";&\" or end window character\n        if (raw_bytes[i] == 59 && raw_bytes[i+1] == 38 && start_idx != -1) { \n            end_idx = i;\n            ch0_val = 0;\n            ch1_val = 0;\n            sign0 = 1;\n            sign1 = 1;\n            phase = 0; \n\n            for (k = start_idx + 1; k < end_idx; k++) {\n                if (raw_bytes[k] == 45) { // '-' sign\n                    if (phase == 0) sign0 = -1;\n                    else sign1 = -1;\n                }\n                else if (raw_bytes[k] == 43) { // '+' sign\n                    if (phase == 0) sign0 = 1;\n                    else sign1 = 1;\n                }\n                else if (raw_bytes[k] == 59) { // ';' delimiter\n                    phase = 1; \n                }\n                else if (raw_bytes[k] >= 48 && raw_bytes[k] <= 57) { // Numeric ASCII digits\n                    if (phase == 0) {\n                        ch0_val = (ch0_val * 10) + (raw_bytes[k] - 48);\n                    } else {\n                        ch1_val = (ch1_val * 10) + (raw_bytes[k] - 48);\n                    }\n                }\n            }\n\n            // Implicit type conversion\n            ch0_raw = ch0_val * sign0 * 1.0;\n            ch1_raw = ch1_val * sign1 * 1.0;\n\n            // FIX: Sanity check / Hard-clamping to catch sudden massive ASCII noise spikes\n            if (ch0_raw > max_allowed_bits)  ch0_raw = max_allowed_bits;\n            if (ch0_raw < -max_allowed_bits) ch0_raw = -max_allowed_bits;\n            if (ch1_raw > max_allowed_bits)  ch1_raw = max_allowed_bits;\n            if (ch1_raw < -max_allowed_bits) ch1_raw = -max_allowed_bits;\n\n            // --- STEP 2: 3-SAMPLE MEDIAN FILTER ---\n            m0_2 = m0_1; m0_1 = m0_0; m0_0 = ch0_raw;\n            float s0_0 = m0_0; float s0_1 = m0_1; float s0_2 = m0_2;\n            if (s0_0 > s0_1) { temp0 = s0_0; s0_0 = s0_1; s0_1 = temp0; }\n            if (s0_1 > s0_2) { temp0 = s0_1; s0_1 = s0_2; s0_2 = temp0; }\n            if (s0_0 > s0_1) { temp0 = s0_0; s0_0 = s0_1; s0_1 = temp0; }\n            ch0_clean = s0_1;\n\n            m1_2 = m1_1; m1_1 = m1_0; m1_0 = ch1_raw;\n            float s1_0 = m1_0; float s1_1 = m1_1; float s1_2 = m1_2;\n            if (s1_0 > s1_1) { temp1 = s1_0; s1_0 = s1_1; s1_1 = temp1; }\n            if (s1_1 > s1_2) { temp1 = s1_1; s1_1 = s1_2; s1_2 = temp1; }\n            if (s1_0 > s1_1) { temp1 = s1_0; s1_0 = s1_1; s1_1 = temp1; }\n            ch1_clean = s1_1;\n\n            // --- STEP 3: EXPONENTIAL FILTER (STREAM LEVEL) ---\n            if (ch0_filt == 0.0) ch0_filt = ch0_clean;\n            if (ch1_filt == 0.0) ch1_filt = ch1_clean;\n\n            ch0_filt = ch0_filt + (ch0_clean - ch0_filt) * 0.125;\n            ch1_filt = ch1_filt + (ch1_clean - ch1_filt) * 0.125;\n\n            // --- STEP 4: MIN/MAX WINDOW CONTINUOUS ACCUMULATION ---\n            if (ch0_filt > max_ch0) max_ch0 = ch0_filt;\n            if (ch0_filt < min_ch0) min_ch0 = ch0_filt;\n            if (ch1_filt > max_ch1) max_ch1 = ch1_filt;\n            if (ch1_filt < min_ch1) min_ch1 = ch1_filt;\n\n            valid_samples++; // FIX: Successfully parsed and accumulated a clean point\n            start_idx = -1; \n        }\n    }\n}\n\n// --- STEP 5: WINDOW EVALUATION ENGINE ---\n// FIX: Condition updated to verify that valid samples exist for both channels\nif (((current_time_ms - start_time_ms) >= 50) && (valid_samples > 0) && (min_ch0 < 9000000.0) && (min_ch1 < 9000000.0)) {\n    window_ready = 1;\n\n    // Linear Bit-to-Voltage Transformations (LVDT - Channel 0)\n    out_LVDT_Min_V = (min_ch0 * VREF) / 8388607.0;\n    out_LVDT_Max_V = (max_ch0 * VREF) / 8388607.0;\n    raw_p2p_v = out_LVDT_Max_V - out_LVDT_Min_V;\n\n    // Linear Bit-to-Voltage Transformations (Piezo - Channel 1)\n    piezo_min_v = (min_ch1 * VREF) / 8388607.0;\n    piezo_max_v = (max_ch1 * VREF) / 8388607.0;\n    \n    // Assign Peak-to-Peak Voltage directly to output indicator (Matches Python logic)\n    out_Piezo_P2P = piezo_max_v - piezo_min_v;\n    \n    // Force scaling calculations using Voltage delta * Newtons/Volt Factor\n    raw_friction = out_Piezo_P2P * PIEZO_CAL_FACTOR ;\n    raw_cof = raw_friction / NORMAL_FORCE;\n\n    // --- STEP 6: OUTPUT METRIC SMOOTHING (Low-Pass Filter Alpha = 0.05) ---\n    // Seed initial historical metrics if first loop iteration\n    if (hist_LVDT_P2P == 0.0) hist_LVDT_P2P = raw_p2p_v;\n    if (hist_Friction == 0.0) hist_Friction = raw_friction;\n    if (hist_COF == 0.0)      hist_COF = raw_cof;\n\n    // Apply exponential output dampening\n    hist_LVDT_P2P = hist_LVDT_P2P + (raw_p2p_v - hist_LVDT_P2P) * 0.05;\n    hist_Friction = hist_Friction + (raw_friction - hist_Friction) * 0.05; // Note: Can drop to 0.02 for more aggressive damping\n    hist_COF      = hist_COF + (raw_cof - hist_COF) * 0.05;\n\n    // Direct smoothed parameters out to UI Indicators\n    out_LVDT_P2P_V = hist_LVDT_P2P;\n    out_Friction_N = hist_Friction;\n    out_COF        = hist_COF;\n\n    // Reset tracking targets to extreme boundaries safely\n    min_ch0 = 9999999.0;\n    max_ch0 = -9999999.0;\n    min_ch1 = 9999999.0;\n    max_ch1 = -9999999.0;\n\n    valid_samples = 0; // FIX: Reset counter for next time frame\n    start_time_ms = current_time_ms;\n}"("raw_bytes"=w2043, "array_size"=w2042, "VREF"="VREF", "PIEZO_CAL_FACTOR"="PIEZO_CAL_FACTOR", "NORMAL_FORCE"="NORMAL_FORCE", "min_ch0"=w2038, "max_ch0"=w2037, "min_ch1"=w2036, "max_ch1"=w2035, "current_time_ms"=w2030, "start_time_ms"=w2029, "ch0_filt"=w2027, "ch1_filt"=w2026, "m0_0"=w2023, "m0_1"=w2022, "m0_2"=w2021, "m1_0"=w2020, "m1_1"=w2019, "m1_2"=w2018, "in_LVDT_Min_V"=w2011, "in_LVDT_Max_V"=w2004, "in_LVDT_P2P_V"=w2003, "in_Piezo_P2P"=w2002, "in_Friction_N"=w2001, "in_COF"=w2000, "hist_LVDT_P2P"=w1998, "hist_Friction"=w1997, "hist_COF"=w1996) -> ("window_ready"=→"Valid_data":dbl, "out_LVDT_Min_V"=w2010:dbl, "out_LVDT_Max_V"=w2009:dbl, "out_LVDT_P2P_V"=w2008:dbl, "out_Piezo_P2P"=w2007:dbl, "out_Friction_N"=w2006:dbl, "out_COF"=w2005:dbl, "min_ch0"=w2034:dbl, "max_ch0"=w2033:dbl, "min_ch1"=w2032:dbl, "max_ch1"=w2031:dbl, "start_time_ms"=w2028:u32, "ch0_filt"=w2025:dbl, "ch1_filt"=w2024:dbl, "m0_0"=w2017:dbl, "m0_1"=w2016:dbl, "m0_2"=w2015:dbl, "m1_0"=w2014:dbl, "m1_1"=w2013:dbl, "m1_2"=w2012:dbl, "hist_LVDT_P2P"=w1995:dbl, "hist_Friction"=w1994:dbl, "hist_COF"=w1993:dbl)
            "LVDT MIN" <- w2010
            "LVDT MAX" <- w2009
            "LVDT Peak" <- w2008
            "pizo raw" <- w2007
            "cof" <- w2005
            "Frictioin Force Raw" <- w2006
          }
        }
      }
      frame Error {
      }
    }
    n1739 = local read "Quit"() -> (w1924:bool)
  }
  n1740 = disable-structure shown="Disabled" {
    disable-tunnel: errorcluster {"status"=TRUE, "code"=0, "source"="Init"} ("error IO") -> [w2069 _]
    disable-tunnel: [w2067 _] -> w47
    frame Disabled {
      n1741 = while {
        shift-right: [w2085] -> w2071
        shift-left: _ -> [w2076]
        shift-right: [w2084] -> w2070
        shift-left: w2069 -> [w2078]
        tunnel: [w2073] -> w2067
        tunnel: [w2083] -> _
        i -> [w2083]
        stop <- w2073 stop-if-true
        n1742 = local read "Port 1a"() -> (w2079:bool)
        n1743 = local read "Port 3"() -> (w2080:bool)
        n1744 = local read "Com Port 1"() -> (w2077:refnum<visa-resource-name>)
        n1745 = Or(x=w2080, y=w2079) -> (x .or. y?=w2082:bool)
        n1746 = Unbundle(w2078) -> ("status"=→"Port 3":bool)  [unwired: 2 out]
        n1747 = Not Equal?(x=w2077, y=w2076) -> (x != y?=w2074:bool)
        n1748 = case shown="True" w2082 {
          frame False {
            w2088 = TRUE ("Visible")
            n1749 = property on="Port 1a" class="Bool (strict)"("Visible"=w2088) -> ()  [unwired: 2 in, 2 out]
            n1750 = property on="Port 3" class="Bool (strict)"("Visible"=w2088) -> ()  [unwired: 2 in, 2 out]
          }
          frame True {
            w2089 = TRUE ("Visible")
            n1751 = property on="Port 1a" class="Bool (strict)"("Visible"=w2089) -> ()  [unwired: 2 in, 2 out]